vi "生产者消费者.vi"() -> ()   [LabVIEW 2013]
doc: "该模板用于创建生产者／消费者模式的应用程序，以事件驱动的方式，生成队列中的项。如需通过响应事件实现代码的异步执行，同时不影响用户界面的响应速度，可考虑用该模式替代“用户界面事件处理器”模式。"
uses:
  <vilib>/Utility/miscctls.llb/LVPositionTypeDef.ctl
panel:
  out "怪物行走":i32(slide) scale=0.0..100.0
  out "人物行走":i32(slide) scale=0.0..100.0
  in  "疾风术簇":T1
  in  "凝冰术簇":T2
  in  "火爪术簇":T3
  in  "怪物":bool=TRUE
  in  "普通攻击簇":T4
  in  "逃跑成功":bool
  in  "龙蟠雕玉":cluster{"琉璃法珠":bool, "介绍框":bool, "剩余":dbl}
  in  "集气攻击簇":T5
  in  "待机":bool
  in  "神":i32(slide) scale=0.0..200.0
  out "沈欺霜":i32(slide) scale=0.0..200.0
  in  "琉璃法珠簇":cluster{"琉璃法珠":bool, "介绍框":bool, "剩余":dbl}
  in  "确定按钮 2":bool
  in  "仙术簇":T6
  in  "物品簇":cluster{"止血草":bool, "鼠儿果":bool, "物品中的放弃":bool}
  out "位置":T7
  in  "定位":bool
  out "集气攻击待机动作":bool
  in  "攻击簇":cluster{"普通攻击":bool, "集气攻击":bool, "攻击中的放弃":bool}
  in  "逃跑":bool
  in  "物品":bool
  in  "仙术":bool
  in  "攻击":bool
  in  "五个状态":enum16{"逃跑", "初始化", "物品", "仙术", "攻击"}(ring)
  # "框图坐标\n207,421,460，498\n沈欺霜坐标\n800,388"
  # "剩余"
  # "个"
  # "剩余"
  # "个"
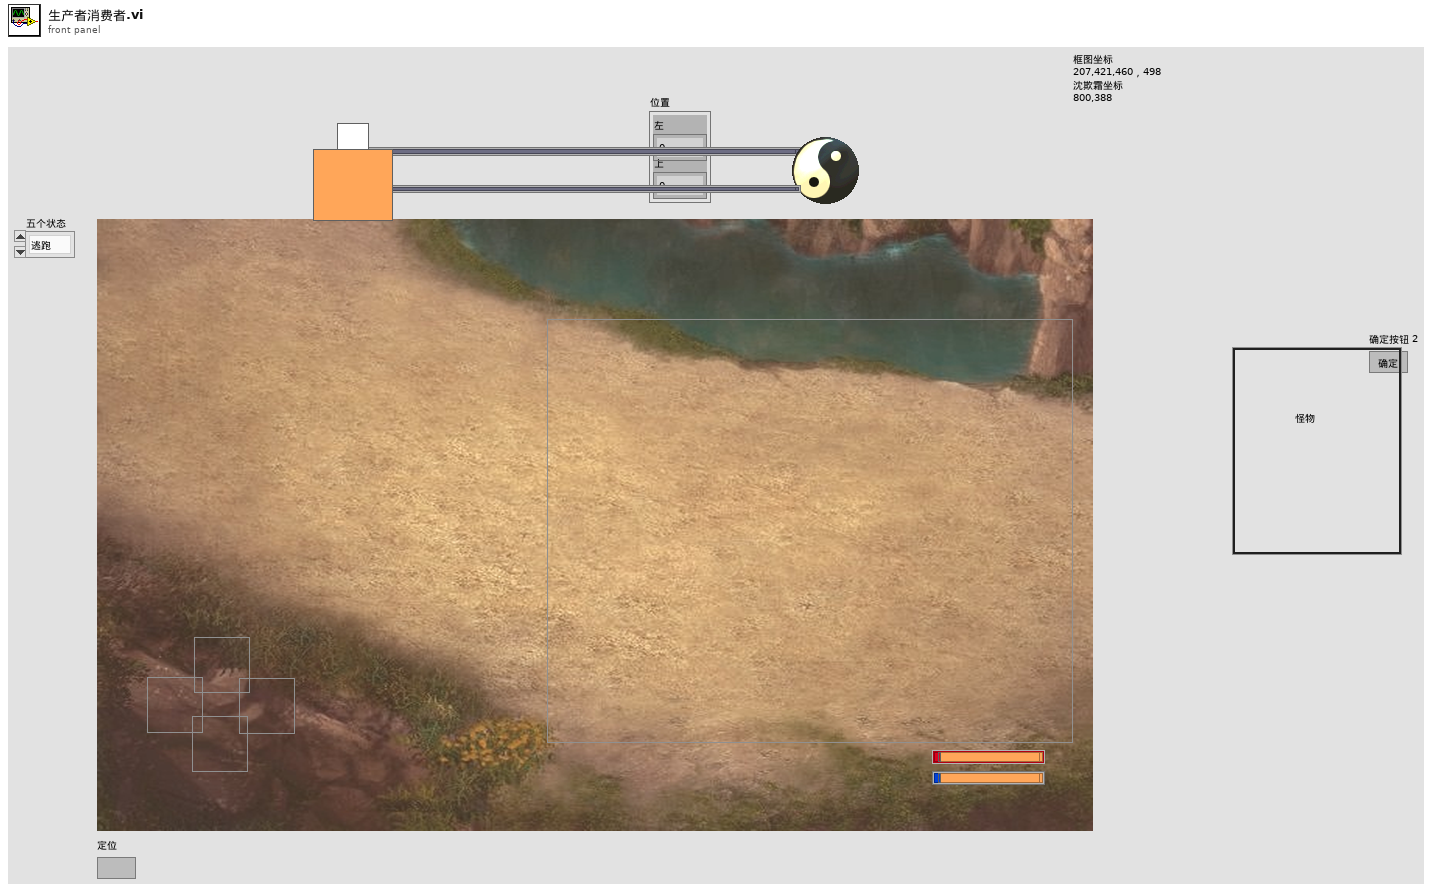
[diagram p1: front panel]
types:
  T1 = cluster{"确定按钮":bool, "确定按钮 2":bool, "确定按钮 3":bool, "确定按钮 4":bool, "确定按钮 5":bool, "确定按钮 6":bool, "确定按钮 7":bool, "确定按钮 8":bool, "确定按钮 9":bool, "确定按钮 10":bool, "确定按钮 11":bool, "确定按钮 12":bool, "确定按钮 13":bool, "确定按钮 14":bool, "确定按钮 15":bool}
  T2 = cluster{"确定按钮1":bool, "确定按钮 2":bool, "确定按钮 3":bool, "确定按钮 4":bool, "确定按钮 5":bool, "确定按钮 6":bool, "确定按钮 7":bool, "确定按钮 8":bool, "确定按钮 9":bool, "确定按钮 10":bool, "确定按钮 11":bool, "确定按钮 12":bool, "确定按钮 13":bool, "确定按钮 14":bool, "确定按钮 15":bool, bool}
  T3 = cluster{"4":bool, "5":bool, "6":bool, "7":bool, "8":bool, "1":bool, "2":bool, "3":bool, "9":bool, "10":bool, "11":bool, "12":bool, "13":bool, "14":bool, "15":bool, "确定按钮":bool}
  T4 = cluster{"1":bool, "2":bool, "3":bool, "4":bool, "5":bool, "6":bool, "7":bool, "8":bool, "9":bool, "减50":bool}
  T5 = cluster{"1":bool, "2":bool, "3":bool, "4":bool, "5":bool, "6":bool, "7":bool, "8":bool, "9":bool, "10":bool, "11":bool, "12":bool, "13":bool, "14":bool, "15":bool, "16":bool, "17":bool}
  T6 = cluster{"火爪术":bool, "凝冰术":bool, "疾风术":bool, "仙术中的放弃":bool}
  T7 = typedef "LVPositionTypeDef.ctl" = cluster{"Left":i32, "Top":i32}
  T8 = cluster{"1":bool, "2":bool, "3":bool, "4":bool, "5":bool, "6":bool, "7":bool, "8":bool, "9":bool}
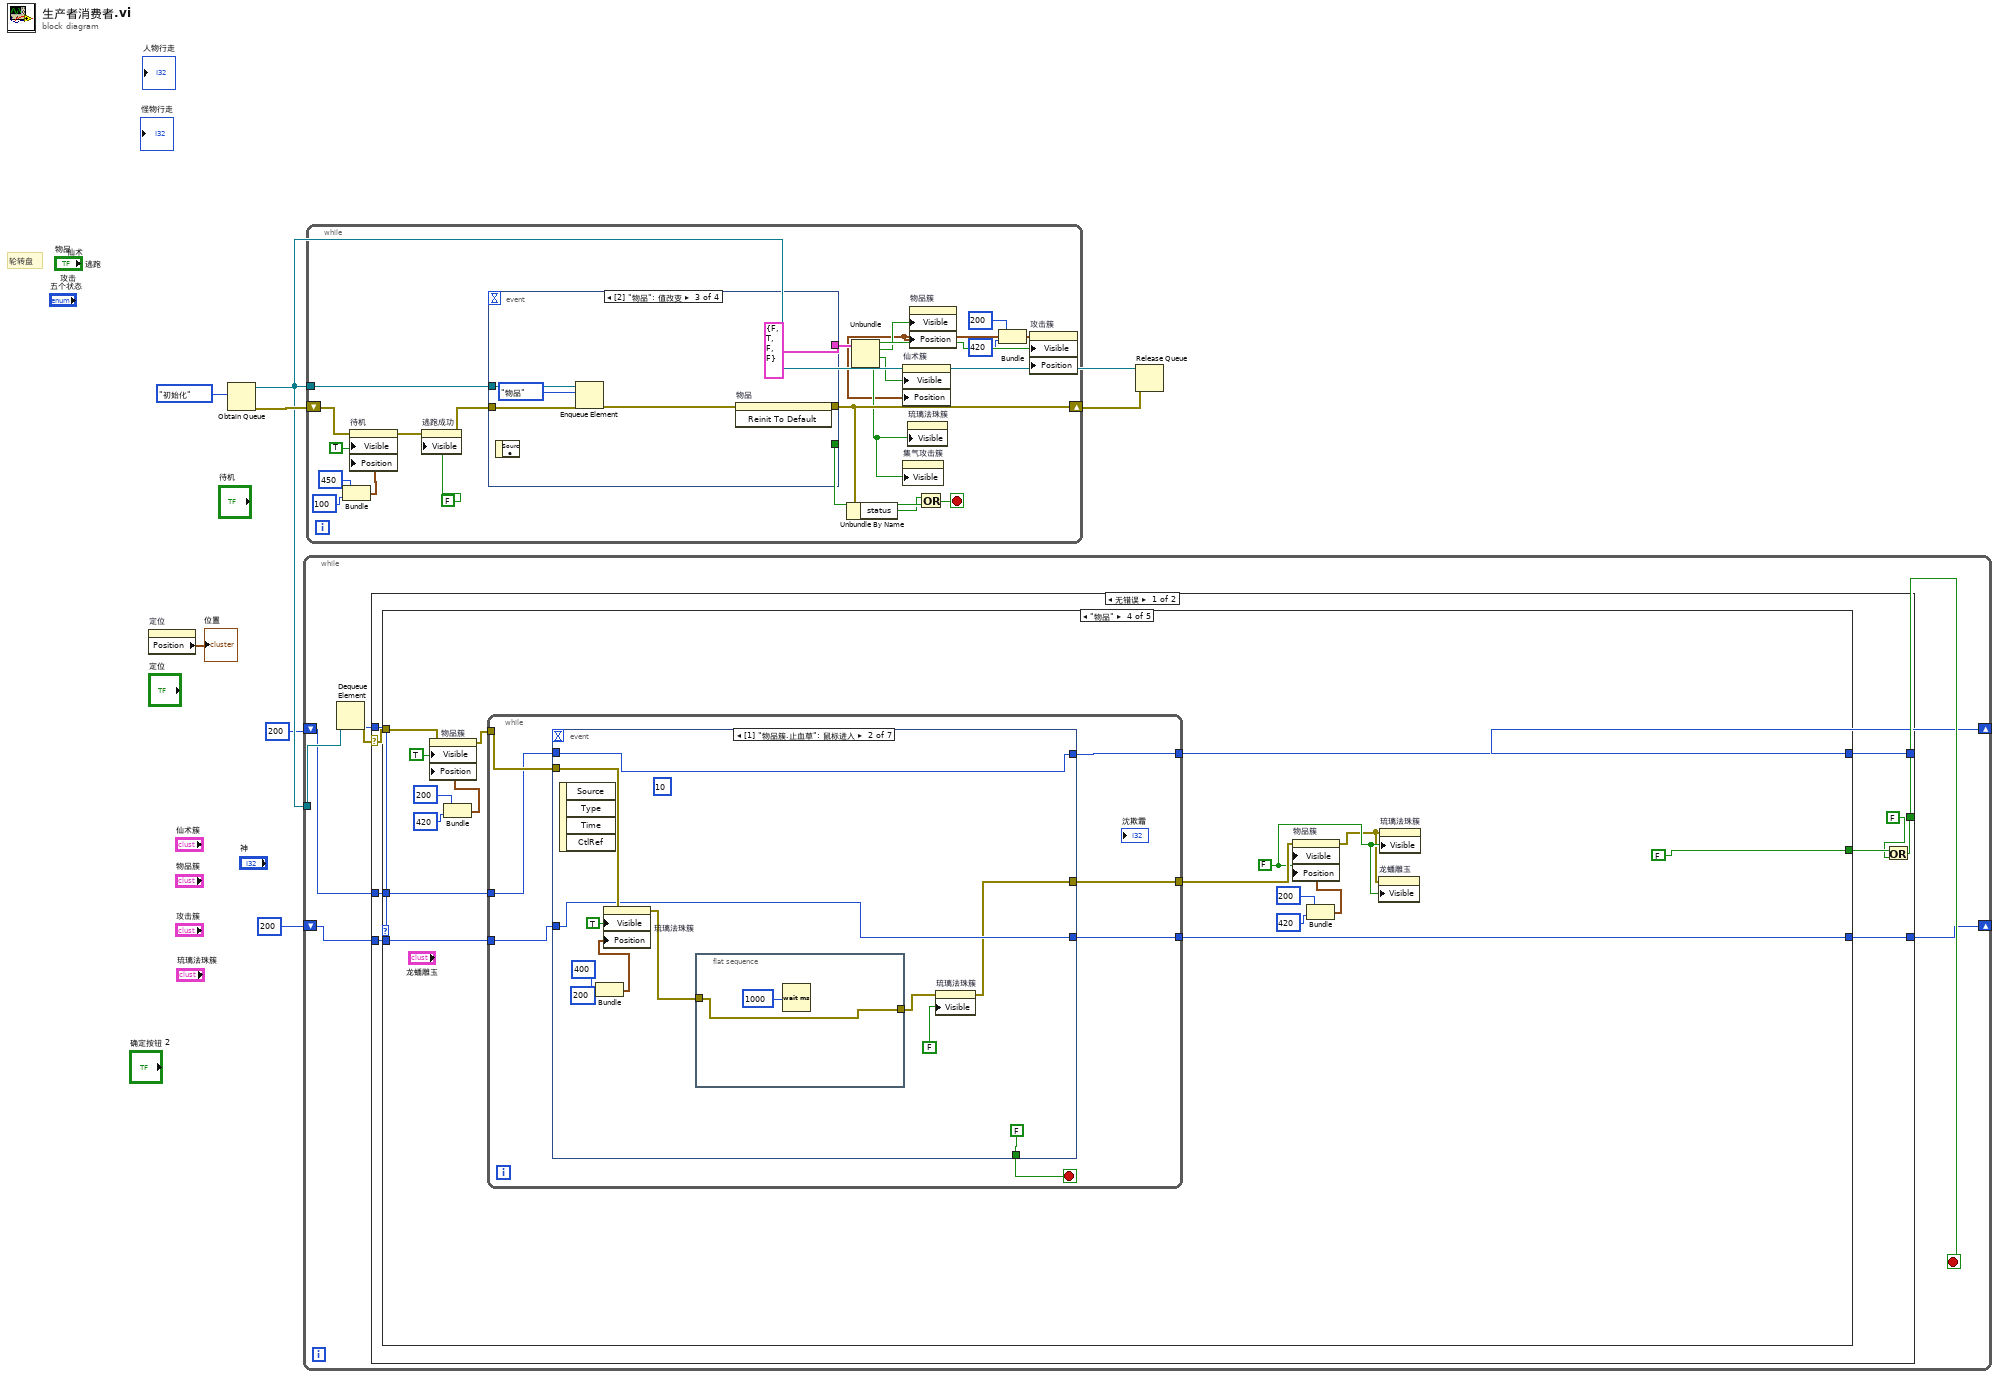
[diagram p0: block diagram]
diagram:
  # "轮转盘"
  n1 = property on="定位" class="Bool"() -> ("Position"=→"位置":T7)  [unwired: 2 in, 2 out]
  n2 = Obtain Queue(element data type=enum16{"逃跑", "初始化", "物品", "仙术", "攻击"}."初始化" ("五个状态")) -> (queue out=w5:refnum<queue>, error out=w7:errorcluster)  [unwired: 4 in, 1 out]
  n3 = while {
    tunnel: w5 -> [w15]
    shift-right: [w10] -> _
    shift-left: 200 -> [w11]
    shift-right: [w8] -> _
    shift-left: 200 -> [w9]
    stop <- w12 stop-if-true
    n4 = Dequeue Element(queue=w15) -> (element=w13:enum16{"逃跑", "初始化", "物品", "仙术", "攻击"}, error out=w14:errorcluster)  [unwired: 2 in, 2 out]
    n5 = case shown="无错误" w14 {
      selector: w14 -> [w23 _]
      tunnel: w13 -> [w24 _]
      tunnel: [w16 TRUE] -> w12
      tunnel: w11 -> [w22 w460]
      tunnel: [w21 w460] -> w10
      tunnel: w9 -> [w20 w459]
      tunnel: [w19 w459] -> w8
      frame No Error {
        n6 = case shown="\"物品\"" w24 {
          tunnel: w23 -> [_ w36 w177 w379 w454]
          tunnel: w22 -> [w27 w30 w175 w374 w453]
          tunnel: [w27 w30 w175 w373 w453] -> w21
          tunnel: w20 -> [w26 w29 w174 w368 w452]
          tunnel: [w26 w29 w174 w367 w452] -> w19
          tunnel: [FALSE FALSE FALSE FALSE w447] -> w18
          frame "初始化", Default {
          }
          frame "攻击" {
            n7 = Bundle(200, 420) -> (w31:cluster{i32, i32})  [unwired: 1 in]
            n8 = property on="攻击簇" class="Clust"(error in=w36, "Visible"=TRUE, "Position"=w31) -> (error out=w34:errorcluster)  [unwired: 1 in, 1 out]
            n9 = while {
              tunnel: w34 -> [w39]
              stop <- w40 stop-if-true
              n10 = event shown="[2] \"攻击簇.攻击中的放弃\": 值改变" {
                selector: _ -> [_ _ _ _]
                dyn-events: _ -> [_ _ _ _]
                timeout: _ -> [_ _ _ _]
                tunnel: [w41 w43 w122 w125] -> w38
                tunnel: [FALSE TRUE TRUE TRUE] -> w40
                tunnel: w39 -> [w41 w49 w122 w137]
                event Timeout {
                  n11 = event-data() -> ()  [unwired: 1 in, 3 out]
                }
                event "攻击簇.集气攻击": Value Change {
                  w58 = TRUE ("可见")
                  n12 = event-data() -> ()  [unwired: 1 in, 6 out]
                  n13 = Bundle(450, 100) -> (w63:cluster{i32, i32})  [unwired: 1 in]
                  n14 = property on="待机" class="Bool"(error in=w49, "Visible"=FALSE) -> (error out=w50:errorcluster)  [unwired: 1 in, 1 out]
                  n15 = property on="攻击簇" class="Clust"(error in=w50, "Visible"=FALSE) -> (error out=w57:errorcluster)  [unwired: 1 in, 1 out]
                  n16 = property on="集气攻击待机动作" class="Bool"(error in=w57, "Position"=w63, "Visible"=w58) -> (error out=w66:errorcluster)  [unwired: 1 in, 1 out]
                  n17 = property on="集气攻击簇" class="Clust"(error in=w57, "Visible"=w58) -> (error out=w56:errorcluster)  [unwired: 1 in, 1 out]
                  n18 = for {
                    N: 20 -> [_]
                    shift-right: [w114] -> _
                    shift-left: _ -> [_]
                    tunnel: w66 -> [w115]
                    tunnel: [w115] -> w61
                    i -> [w116]
                    n19 = Quotient & Remainder(x=w116, y=2) -> (x-y*floor(x/y)=w118:i32)  [unwired: 1 out]
                    n20 = case shown="1" w118 {
                      tunnel: [TRUE FALSE] -> w114
                      frame 0, Default {
                      }
                      frame 1 {
                      }
                    }
                    "集气攻击待机动作" <- w114
                    n21 = Wait (ms)(milliseconds to wait=u32 100 ("等待时间（毫秒）")) -> ()  [unwired: 1 out]
                  }
                  n22 = while {
                    tunnel: w56 -> [w68]
                    tunnel: [w68] -> w55
                    stop <- w69 stop-if-true
                    n23 = flat-sequence {
                      tunnel: [TRUE] -> w69
                      frame #0 {
                        n24 = for {
                          N: 17 -> [_]
                          i -> [w81]
                          n25 = Wait (ms)(milliseconds to wait=100) -> ()  [unwired: 1 out]
                          n26 = case shown="0, 默认" w81 {
                            tunnel: [T5 {"1"=TRUE, "2"=FALSE, "3"=FALSE, "4"=FALSE, "5"=FALSE, "6"=FALSE, "7"=FALSE, "8"=FALSE, "9"=FALSE, "10"=FALSE, "11"=FALSE, "12"=FALSE, "13"=FALSE, "14"=FALSE, "15"=FALSE, "16"=FALSE, "17"=FALSE} ("簇") T5 {"1"=FALSE, "2"=TRUE, "3"=FALSE, "4"=FALSE, "5"=FALSE, "6"=FALSE, "7"=FALSE, "8"=FALSE, "9"=FALSE, "10"=FALSE, "11"=FALSE, "12"=FALSE, "13"=FALSE, "14"=FALSE, "15"=FALSE, "16"=FALSE, "17"=FALSE} ("簇") T5 {"1"=FALSE, "2"=FALSE, "3"=TRUE, "4"=FALSE, "5"=FALSE, "6"=FALSE, "7"=FALSE, "8"=FALSE, "9"=FALSE, "10"=FALSE, "11"=FALSE, "12"=FALSE, "13"=FALSE, "14"=FALSE, "15"=FALSE, "16"=FALSE, "17"=FALSE} ("簇") T5 {"1"=FALSE, "2"=FALSE, "3"=FALSE, "4"=TRUE, "5"=FALSE, "6"=FALSE, "7"=FALSE, "8"=FALSE, "9"=FALSE, "10"=FALSE, "11"=FALSE, "12"=FALSE, "13"=FALSE, "14"=FALSE, "15"=FALSE, "16"=FALSE, "17"=FALSE} ("簇") T5 {"1"=FALSE, "2"=FALSE, "3"=FALSE, "4"=FALSE, "5"=TRUE, "6"=FALSE, "7"=FALSE, "8"=FALSE, "9"=FALSE, "10"=FALSE, "11"=FALSE, "12"=FALSE, "13"=FALSE, "14"=FALSE, "15"=FALSE, "16"=FALSE, "17"=FALSE} ("簇") T5 {"1"=FALSE, "2"=FALSE, "3"=FALSE, "4"=FALSE, "5"=FALSE, "6"=TRUE, "7"=FALSE, "8"=FALSE, "9"=FALSE, "10"=FALSE, "11"=FALSE, "12"=FALSE, "13"=FALSE, "14"=FALSE, "15"=FALSE, "16"=FALSE, "17"=FALSE} ("簇") T5 {"1"=FALSE, "2"=FALSE, "3"=FALSE, "4"=FALSE, "5"=FALSE, "6"=FALSE, "7"=TRUE, "8"=FALSE, "9"=FALSE, "10"=FALSE, "11"=FALSE, "12"=FALSE, "13"=FALSE, "14"=FALSE, "15"=FALSE, "16"=FALSE, "17"=FALSE} ("簇") T5 {"1"=FALSE, "2"=FALSE, "3"=FALSE, "4"=FALSE, "5"=FALSE, "6"=FALSE, "7"=FALSE, "8"=TRUE, "9"=FALSE, "10"=FALSE, "11"=FALSE, "12"=FALSE, "13"=FALSE, "14"=FALSE, "15"=FALSE, "16"=FALSE, "17"=FALSE} ("簇") T5 {"1"=FALSE, "2"=FALSE, "3"=FALSE, "4"=FALSE, "5"=FALSE, "6"=FALSE, "7"=FALSE, "8"=FALSE, "9"=TRUE, "10"=FALSE, "11"=FALSE, "12"=FALSE, "13"=FALSE, "14"=FALSE, "15"=FALSE, "16"=FALSE, "17"=FALSE} ("簇") T5 {"1"=FALSE, "2"=FALSE, "3"=FALSE, "4"=FALSE, "5"=FALSE, "6"=FALSE, "7"=FALSE, "8"=FALSE, "9"=FALSE, "10"=TRUE, "11"=FALSE, "12"=FALSE, "13"=FALSE, "14"=FALSE, "15"=FALSE, "16"=FALSE, "17"=FALSE} ("簇") T5 {"1"=FALSE, "2"=FALSE, "3"=FALSE, "4"=FALSE, "5"=FALSE, "6"=FALSE, "7"=FALSE, "8"=FALSE, "9"=FALSE, "10"=FALSE, "11"=TRUE, "12"=FALSE, "13"=FALSE, "14"=FALSE, "15"=FALSE, "16"=FALSE, "17"=FALSE} ("簇") T5 {"1"=FALSE, "2"=FALSE, "3"=FALSE, "4"=FALSE, "5"=FALSE, "6"=FALSE, "7"=FALSE, "8"=FALSE, "9"=FALSE, "10"=FALSE, "11"=FALSE, "12"=TRUE, "13"=FALSE, "14"=FALSE, "15"=FALSE, "16"=FALSE, "17"=FALSE} ("簇") T5 {"1"=FALSE, "2"=FALSE, "3"=FALSE, "4"=FALSE, "5"=FALSE, "6"=FALSE, "7"=FALSE, "8"=FALSE, "9"=FALSE, "10"=FALSE, "11"=FALSE, "12"=FALSE, "13"=TRUE, "14"=FALSE, "15"=FALSE, "16"=FALSE, "17"=FALSE} ("簇") T5 {"1"=FALSE, "2"=FALSE, "3"=FALSE, "4"=FALSE, "5"=FALSE, "6"=FALSE, "7"=FALSE, "8"=FALSE, "9"=FALSE, "10"=FALSE, "11"=FALSE, "12"=FALSE, "13"=FALSE, "14"=TRUE, "15"=FALSE, "16"=FALSE, "17"=FALSE} ("簇") T5 {"1"=FALSE, "2"=FALSE, "3"=FALSE, "4"=FALSE, "5"=FALSE, "6"=FALSE, "7"=FALSE, "8"=FALSE, "9"=FALSE, "10"=FALSE, "11"=FALSE, "12"=FALSE, "13"=FALSE, "14"=FALSE, "15"=TRUE, "16"=FALSE, "17"=FALSE} ("簇") T5 {"1"=FALSE, "2"=FALSE, "3"=FALSE, "4"=FALSE, "5"=FALSE, "6"=FALSE, "7"=FALSE, "8"=FALSE, "9"=FALSE, "10"=FALSE, "11"=FALSE, "12"=FALSE, "13"=FALSE, "14"=FALSE, "15"=FALSE, "16"=TRUE, "17"=FALSE} ("簇") T5 {"1"=FALSE, "2"=FALSE, "3"=FALSE, "4"=FALSE, "5"=FALSE, "6"=FALSE, "7"=FALSE, "8"=FALSE, "9"=FALSE, "10"=FALSE, "11"=FALSE, "12"=FALSE, "13"=FALSE, "14"=FALSE, "15"=FALSE, "16"=FALSE, "17"=TRUE} ("簇")] -> w80
                            frame 0, Default {
                            }
                            frame 1 {
                            }
                            frame 2 {
                            }
                            frame 3 {
                            }
                            frame 4 {
                            }
                            frame 5 {
                            }
                            frame 6 {
                            }
                            frame 7 {
                            }
                            frame 8 {
                            }
                            frame 9 {
                            }
                            frame 10 {
                            }
                            frame 11 {
                            }
                            frame 12 {
                            }
                            frame 13 {
                            }
                            frame 14 {
                            }
                            frame 15 {
                            }
                            frame 16 {
                            }
                          }
                          n27 = Unbundle(w80) -> ("1"=w92:bool, "2"=w91:bool, "3"=w90:bool, "4"=w89:bool, "5"=w88:bool, "6"=w87:bool, "7"=w86:bool, "8"=w85:bool, "9"=w82:bool, "10"=w79:bool, "11"=w78:bool, "12"=w77:bool, "13"=w76:bool, "14"=w75:bool, "15"=w74:bool, "16"=w73:bool, "17"=w72:bool)
                          n28 = Bundle(0, -50) -> (w71:cluster{i32, i32})  [unwired: 1 in]
                          n29 = property on="10" class="Bool"("Visible"=w79, "Position"=w71) -> ()  [unwired: 2 in, 2 out]
                          n30 = property on="5" class="Bool"("Visible"=w88, "Position"=w71) -> ()  [unwired: 2 in, 2 out]
                          n31 = property on="14" class="Bool"("Visible"=w75, "Position"=w71) -> ()  [unwired: 2 in, 2 out]
                          n32 = property on="1" class="Bool"("Visible"=w92, "Position"=w71) -> ()  [unwired: 2 in, 2 out]
                          n33 = property on="6" class="Bool"("Visible"=w87, "Position"=w71) -> ()  [unwired: 2 in, 2 out]
                          n34 = property on="11" class="Bool"("Visible"=w78, "Position"=w71) -> ()  [unwired: 2 in, 2 out]
                          n35 = property on="2" class="Bool"("Visible"=w91, "Position"=w71) -> ()  [unwired: 2 in, 2 out]
                          n36 = property on="15" class="Bool"("Visible"=w74, "Position"=w71) -> ()  [unwired: 2 in, 2 out]
                          n37 = property on="7" class="Bool"("Visible"=w86, "Position"=w71) -> ()  [unwired: 2 in, 2 out]
                          n38 = property on="3" class="Bool"("Visible"=w90, "Position"=w71) -> ()  [unwired: 2 in, 2 out]
                          n39 = property on="12" class="Bool"("Visible"=w77, "Position"=w71) -> ()  [unwired: 2 in, 2 out]
                          n40 = property on="8" class="Bool"("Visible"=w85, "Position"=w71) -> ()  [unwired: 2 in, 2 out]
                          n41 = property on="4" class="Bool"("Visible"=w89, "Position"=w71) -> ()  [unwired: 2 in, 2 out]
                          n42 = property on="16" class="Bool"("Visible"=w73, "Position"=w71) -> ()  [unwired: 2 in, 2 out]
                          n43 = property on="13" class="Bool"("Visible"=w76, "Position"=w71) -> ()  [unwired: 2 in, 2 out]
                          n44 = property on="9" class="Bool"("Visible"=w82, "Position"=w71) -> ()  [unwired: 2 in, 2 out]
                          n45 = property on="17" class="Bool"("Visible"=w72, "Position"=w71) -> ()  [unwired: 2 in, 2 out]
                        }
                      }
                      frame #1 {
                        n46 = Wait (ms)(milliseconds to wait=500) -> ()  [unwired: 1 out]
                      }
                      frame #2 {
                        n47 = property on="17" class="Bool"("Visible"=FALSE) -> ()  [unwired: 2 in, 2 out]
                      }
                    }
                  }
                  n48 = property on="集气攻击待机动作" class="Bool"(error in=w61, "Visible"=FALSE) -> (error out=w53:errorcluster)  [unwired: 1 in, 1 out]
                  n49 = property on="集气攻击簇" class="Clust"(error in=w55, "Visible"=FALSE) -> (error out=w52:errorcluster)  [unwired: 1 in, 1 out]
                  n50 = Bundle(450, 100) -> (w46:cluster{i32, i32})  [unwired: 1 in]
                  n51 = Merge Errors(w53, w52) -> (w44:errorcluster)
                  n52 = property on="待机" class="Bool"(error in=w44, "Visible"=TRUE, "Position"=w46) -> (error out=w43:errorcluster)  [unwired: 1 in, 1 out]
                }
                event "攻击簇.攻击中的放弃": Value Change {
                  n53 = event-data() -> ()  [unwired: 1 in, 6 out]
                }
                event "攻击簇.普通攻击": Value Change {
                  n54 = event-data() -> ()  [unwired: 1 in, 6 out]
                  n55 = Bundle(0, 0) -> (w132:cluster{i32, i32})  [unwired: 1 in]
                  n56 = property on="待机" class="Bool"(error in=w137, "Visible"=FALSE) -> (error out=w136:errorcluster)  [unwired: 1 in, 1 out]
                  n57 = property on="攻击簇" class="Clust"(error in=w136, "Visible"=FALSE) -> (error out=w130:errorcluster)  [unwired: 1 in, 1 out]
                  n58 = property on="普通攻击簇" class="Clust"(error in=w130, "Visible"=TRUE, "Position"=w132) -> (error out=w131:errorcluster)  [unwired: 1 in, 1 out]
                  n59 = while {
                    tunnel: w131 -> [w140]
                    tunnel: [w140] -> w128
                    stop <- w141 stop-if-true
                    n60 = flat-sequence {
                      tunnel: [TRUE] -> w141
                      frame #0 {
                        n61 = for {
                          N: 9 -> [_]
                          i -> [w149]
                          n62 = Wait (ms)(milliseconds to wait=100) -> ()  [unwired: 1 out]
                          n63 = case shown="0, 默认" w149 {
                            tunnel: [T8 {"1"=TRUE, "2"=FALSE, "3"=FALSE, "4"=FALSE, "5"=FALSE, "6"=FALSE, "7"=FALSE, "8"=FALSE, "9"=FALSE} ("簇") T8 {"1"=FALSE, "2"=TRUE, "3"=FALSE, "4"=FALSE, "5"=FALSE, "6"=FALSE, "7"=FALSE, "8"=FALSE, "9"=FALSE} ("簇") T8 {"1"=FALSE, "2"=FALSE, "3"=TRUE, "4"=FALSE, "5"=FALSE, "6"=FALSE, "7"=FALSE, "8"=FALSE, "9"=FALSE} ("簇") T8 {"1"=FALSE, "2"=FALSE, "3"=FALSE, "4"=TRUE, "5"=FALSE, "6"=FALSE, "7"=FALSE, "8"=FALSE, "9"=FALSE} ("簇") T8 {"1"=FALSE, "2"=FALSE, "3"=FALSE, "4"=FALSE, "5"=TRUE, "6"=FALSE, "7"=FALSE, "8"=FALSE, "9"=FALSE} ("簇") T8 {"1"=FALSE, "2"=FALSE, "3"=FALSE, "4"=FALSE, "5"=FALSE, "6"=TRUE, "7"=FALSE, "8"=FALSE, "9"=FALSE} ("簇") T8 {"1"=FALSE, "2"=FALSE, "3"=FALSE, "4"=FALSE, "5"=FALSE, "6"=FALSE, "7"=TRUE, "8"=FALSE, "9"=FALSE} ("簇") T8 {"1"=FALSE, "2"=FALSE, "3"=FALSE, "4"=FALSE, "5"=FALSE, "6"=FALSE, "7"=FALSE, "8"=TRUE, "9"=FALSE} ("簇") T8 {"1"=FALSE, "2"=FALSE, "3"=FALSE, "4"=FALSE, "5"=FALSE, "6"=FALSE, "7"=FALSE, "8"=FALSE, "9"=TRUE} ("簇")] -> w148
                            frame 0, Default {
                            }
                            frame 1 {
                            }
                            frame 2 {
                            }
                            frame 3 {
                            }
                            frame 4 {
                            }
                            frame 5 {
                            }
                            frame 6 {
                            }
                            frame 7 {
                            }
                            frame 8 {
                            }
                          }
                          n64 = Bundle(0, -50) -> (w147:cluster{i32, i32})  [unwired: 1 in]
                          n65 = Unbundle(w148) -> ("1"=w159:bool, "2"=w158:bool, "3"=w157:bool, "4"=w156:bool, "5"=w155:bool, "6"=w154:bool, "7"=w153:bool, "8"=w152:bool, "9"=w146:bool)
                          n66 = property on="5" class="Bool"("Visible"=w155, "Position"=w147) -> ()  [unwired: 2 in, 2 out]
                          n67 = property on="1" class="Bool"("Visible"=w159, "Position"=w147) -> ()  [unwired: 2 in, 2 out]
                          n68 = property on="6" class="Bool"("Visible"=w154, "Position"=w147) -> ()  [unwired: 2 in, 2 out]
                          n69 = property on="2" class="Bool"("Visible"=w158, "Position"=w147) -> ()  [unwired: 2 in, 2 out]
                          n70 = property on="7" class="Bool"("Visible"=w153, "Position"=w147) -> ()  [unwired: 2 in, 2 out]
                          n71 = property on="3" class="Bool"("Visible"=w157, "Position"=w147) -> ()  [unwired: 2 in, 2 out]
                          n72 = property on="8" class="Bool"("Visible"=w152, "Position"=w147) -> ()  [unwired: 2 in, 2 out]
                          n73 = property on="4" class="Bool"("Visible"=w156, "Position"=w147) -> ()  [unwired: 2 in, 2 out]
                          n74 = Bundle(100, 100) -> (w143:cluster{i32, i32})  [unwired: 1 in]
                          n75 = property on="9" class="Bool"("Visible"=w146, "Position"=w147) -> ()  [unwired: 2 in, 2 out]
                          n76 = property on="减50" class="Bool"("Visible"=w146, "Position"=w143) -> ()  [unwired: 2 in, 2 out]
                        }
                      }
                      frame #1 {
                        n77 = Wait (ms)(milliseconds to wait=500) -> ()  [unwired: 1 out]
                      }
                      frame #2 {
                        w172 = FALSE
                        n78 = property on="9" class="Bool"("Visible"=w172) -> ()  [unwired: 2 in, 2 out]
                        n79 = property on="减50" class="Bool"("Visible"=w172) -> ()  [unwired: 2 in, 2 out]
                      }
                    }
                  }
                  n80 = property on="普通攻击簇" class="Clust"(error in=w128, "Visible"=FALSE) -> (error out=w127:errorcluster)  [unwired: 1 in, 1 out]
                  n81 = property on="待机" class="Bool"(error in=w127, "Visible"=TRUE) -> (error out=w125:errorcluster)  [unwired: 1 in, 1 out]
                }
              }
              n82 = property on="攻击簇" class="Clust"(error in=w38, "Visible"=FALSE) -> ()  [unwired: 1 in, 2 out]
            }
          }
          frame "仙术" {
            n83 = Bundle(200, 420) -> (w178:cluster{i32, i32})  [unwired: 1 in]
            n84 = property on="仙术簇" class="Clust"(error in=w177, "Visible"=TRUE, "Position"=w178) -> (error out=w176:errorcluster)  [unwired: 1 in, 1 out]
            n85 = while {
              tunnel: w176 -> [w183]
              stop <- w182 stop-if-true
              n86 = event shown="[4] \"仙术簇.仙术中的放弃\": 值改变" {
                selector: _ -> [_ _ _ _ _]
                dyn-events: _ -> [_ _ _ _ _]
                timeout: _ -> [_ _ _ _ _]
                tunnel: w183 -> [_ w192 w251 w310 w361]
                tunnel: [FALSE TRUE TRUE TRUE TRUE] -> w182
                event Timeout {
                  n87 = event-data() -> ()  [unwired: 1 in, 3 out]
                }
                event "仙术簇.火爪术": Value Change {
                  n88 = event-data() -> ()  [unwired: 1 in, 6 out]
                  n89 = Bundle(0, 0) -> (w189:cluster{i32, i32})  [unwired: 1 in]
                  n90 = property on="仙术簇" class="Clust"(error in=w192, "Visible"=FALSE) -> (error out=w195:errorcluster)  [unwired: 1 in, 1 out]
                  n91 = property on="待机" class="Bool"(error in=w195, "Visible"=TRUE) -> (error out=w193:errorcluster)  [unwired: 1 in, 1 out]
                  n92 = property on="火爪术簇" class="Clust"(error in=w193, "Visible"=TRUE, "Position"=w189) -> (error out=w188:errorcluster)  [unwired: 1 in, 1 out]
                  n93 = while {
                    tunnel: w188 -> [w198]
                    tunnel: [w198] -> w187
                    stop <- w199 stop-if-true
                    n94 = flat-sequence {
                      tunnel: [TRUE] -> w199
                      frame #0 {
                        n95 = for {
                          N: 15 -> [_]
                          i -> [w211]
                          n96 = Wait (ms)(milliseconds to wait=100) -> ()  [unwired: 1 out]
                          n97 = case shown="14" w211 {
                            tunnel: [T3 {"4"=TRUE, "5"=FALSE, "6"=FALSE, "7"=FALSE, "8"=FALSE, "1"=FALSE, "2"=FALSE, "3"=FALSE, "9"=FALSE, "10"=FALSE, "11"=FALSE, "12"=FALSE, "13"=FALSE, "14"=FALSE, "15"=FALSE, "确定按钮"=FALSE} ("簇") T3 {"4"=FALSE, "5"=TRUE, "6"=FALSE, "7"=FALSE, "8"=FALSE, "1"=FALSE, "2"=FALSE, "3"=FALSE, "9"=FALSE, "10"=FALSE, "11"=FALSE, "12"=FALSE, "13"=FALSE, "14"=FALSE, "15"=FALSE, "确定按钮"=FALSE} ("簇") T3 {"4"=FALSE, "5"=FALSE, "6"=TRUE, "7"=FALSE, "8"=FALSE, "1"=FALSE, "2"=FALSE, "3"=FALSE, "9"=FALSE, "10"=FALSE, "11"=FALSE, "12"=FALSE, "13"=FALSE, "14"=FALSE, "15"=FALSE, "确定按钮"=FALSE} ("簇") T3 {"4"=FALSE, "5"=FALSE, "6"=FALSE, "7"=TRUE, "8"=FALSE, "1"=FALSE, "2"=FALSE, "3"=FALSE, "9"=FALSE, "10"=FALSE, "11"=FALSE, "12"=FALSE, "13"=FALSE, "14"=FALSE, "15"=FALSE, "确定按钮"=FALSE} ("簇") T3 {"4"=FALSE, "5"=FALSE, "6"=FALSE, "7"=FALSE, "8"=TRUE, "1"=FALSE, "2"=FALSE, "3"=FALSE, "9"=FALSE, "10"=FALSE, "11"=FALSE, "12"=FALSE, "13"=FALSE, "14"=FALSE, "15"=FALSE, "确定按钮"=FALSE} ("簇") T3 {"4"=FALSE, "5"=FALSE, "6"=FALSE, "7"=FALSE, "8"=FALSE, "1"=TRUE, "2"=FALSE, "3"=FALSE, "9"=FALSE, "10"=FALSE, "11"=FALSE, "12"=FALSE, "13"=FALSE, "14"=FALSE, "15"=FALSE, "确定按钮"=FALSE} ("簇") T3 {"4"=FALSE, "5"=FALSE, "6"=FALSE, "7"=FALSE, "8"=FALSE, "1"=FALSE, "2"=TRUE, "3"=FALSE, "9"=FALSE, "10"=FALSE, "11"=FALSE, "12"=FALSE, "13"=FALSE, "14"=FALSE, "15"=FALSE, "确定按钮"=FALSE} ("簇") T3 {"4"=FALSE, "5"=FALSE, "6"=FALSE, "7"=FALSE, "8"=FALSE, "1"=FALSE, "2"=FALSE, "3"=TRUE, "9"=FALSE, "10"=FALSE, "11"=FALSE, "12"=FALSE, "13"=FALSE, "14"=FALSE, "15"=FALSE, "确定按钮"=FALSE} ("簇") T3 {"4"=FALSE, "5"=FALSE, "6"=FALSE, "7"=FALSE, "8"=FALSE, "1"=FALSE, "2"=FALSE, "3"=FALSE, "9"=TRUE, "10"=FALSE, "11"=FALSE, "12"=FALSE, "13"=FALSE, "14"=FALSE, "15"=FALSE, "确定按钮"=FALSE} ("簇") T3 {"4"=FALSE, "5"=FALSE, "6"=FALSE, "7"=FALSE, "8"=FALSE, "1"=FALSE, "2"=FALSE, "3"=FALSE, "9"=FALSE, "10"=TRUE, "11"=FALSE, "12"=FALSE, "13"=FALSE, "14"=FALSE, "15"=FALSE, "确定按钮"=FALSE} ("簇") T3 {"4"=FALSE, "5"=FALSE, "6"=FALSE, "7"=FALSE, "8"=FALSE, "1"=FALSE, "2"=FALSE, "3"=FALSE, "9"=FALSE, "10"=FALSE, "11"=TRUE, "12"=FALSE, "13"=FALSE, "14"=FALSE, "15"=FALSE, "确定按钮"=FALSE} ("簇") T3 {"4"=FALSE, "5"=FALSE, "6"=FALSE, "7"=FALSE, "8"=FALSE, "1"=FALSE, "2"=FALSE, "3"=FALSE, "9"=FALSE, "10"=FALSE, "11"=FALSE, "12"=TRUE, "13"=FALSE, "14"=FALSE, "15"=FALSE, "确定按钮"=FALSE} ("簇") T3 {"4"=FALSE, "5"=FALSE, "6"=FALSE, "7"=FALSE, "8"=FALSE, "1"=FALSE, "2"=FALSE, "3"=FALSE, "9"=FALSE, "10"=FALSE, "11"=FALSE, "12"=FALSE, "13"=TRUE, "14"=FALSE, "15"=FALSE, "确定按钮"=FALSE} ("簇") T3 {"4"=FALSE, "5"=FALSE, "6"=FALSE, "7"=FALSE, "8"=FALSE, "1"=FALSE, "2"=FALSE, "3"=FALSE, "9"=FALSE, "10"=FALSE, "11"=FALSE, "12"=FALSE, "13"=FALSE, "14"=TRUE, "15"=FALSE, "确定按钮"=FALSE} ("簇") T3 {"4"=FALSE, "5"=FALSE, "6"=FALSE, "7"=FALSE, "8"=FALSE, "1"=FALSE, "2"=FALSE, "3"=FALSE, "9"=FALSE, "10"=FALSE, "11"=FALSE, "12"=FALSE, "13"=FALSE, "14"=FALSE, "15"=TRUE, "确定按钮"=FALSE} ("簇")] -> w210
                            frame 0, Default {
                            }
                            frame 1 {
                            }
                            frame 2 {
                            }
                            frame 3 {
                            }
                            frame 4 {
                            }
                            frame 5 {
                            }
                            frame 6 {
                            }
                            frame 7 {
                            }
                            frame 8 {
                            }
                            frame 9 {
                            }
                            frame 10 {
                            }
                            frame 11 {
                            }
                            frame 12 {
                            }
                            frame 13 {
                            }
                            frame 14 {
                            }
                          }
                          n98 = Unbundle(w210) -> ("4"=w223:bool, "5"=w222:bool, "6"=w221:bool, "7"=w220:bool, "8"=w219:bool, "1"=w218:bool, "2"=w206:bool, "3"=w205:bool, "9"=w215:bool, "10"=w214:bool, "11"=w209:bool, "12"=w213:bool, "13"=w203:bool, "14"=w204:bool, "15"=w201:bool)  [unwired: 1 out]
                          n99 = Bundle(0, 0) -> (w212:cluster{i32, i32})  [unwired: 1 in]
                          n100 = property on="10" class="Bool"("Visible"=w214, "Position"=w212) -> ()  [unwired: 2 in, 2 out]
                          n101 = property on="14" class="Bool"("Visible"=w204, "Position"=w212) -> ()  [unwired: 2 in, 2 out]
                          n102 = property on="5" class="Bool"("Visible"=w219, "Position"=w212) -> ()  [unwired: 2 in, 2 out]
                          n103 = property on="1" class="Bool"("Visible"=w223, "Position"=w212) -> ()  [unwired: 2 in, 2 out]
                          n104 = property on="6" class="Bool"("Visible"=w218, "Position"=w212) -> ()  [unwired: 2 in, 2 out]
                          n105 = property on="11" class="Bool"("Visible"=w209, "Position"=w212) -> ()  [unwired: 2 in, 2 out]
                          n106 = property on="2" class="Bool"("Visible"=w222, "Position"=w212) -> ()  [unwired: 2 in, 2 out]
                          n107 = property on="15" class="Bool"("Visible"=w201, "Position"=w212) -> ()  [unwired: 2 in, 2 out]
                          n108 = property on="7" class="Bool"("Visible"=w206, "Position"=w212) -> ()  [unwired: 2 in, 2 out]
                          n109 = property on="3" class="Bool"("Visible"=w221, "Position"=w212) -> ()  [unwired: 2 in, 2 out]
                          n110 = property on="12" class="Bool"("Visible"=w213, "Position"=w212) -> ()  [unwired: 2 in, 2 out]
                          n111 = property on="8" class="Bool"("Visible"=w205, "Position"=w212) -> ()  [unwired: 2 in, 2 out]
                          n112 = Bundle(100, 100) -> (w202:cluster{i32, i32})  [unwired: 1 in]
                          n113 = property on="4" class="Bool"("Visible"=w220, "Position"=w212) -> ()  [unwired: 2 in, 2 out]
                          n114 = property on="13" class="Bool"("Visible"=w203, "Position"=w212) -> ()  [unwired: 2 in, 2 out]
                          n115 = property on="确定按钮" class="Bool"("Visible"=w201, "Position"=w202) -> ()  [unwired: 2 in, 2 out]
                          n116 = property on="9" class="Bool"("Visible"=w215, "Position"=w212) -> ()  [unwired: 2 in, 2 out]
                        }
                      }
                      frame #1 {
                        n117 = Wait (ms)(milliseconds to wait=500) -> ()  [unwired: 1 out]